vi "FlexMag - 23-03-2023.vi"() -> ()   [LabVIEW 2018] (continued)
                                n19635 = case shown="False" w23986 {
                                frame False {
                                n19636 = local read "coating start"() -> (w23987:bool)
                                n19637 = case shown="True" w23987 {
                                frame False {
                                }
                                frame True {
                                n19638 = while {
                                i -> [w23990]
                                stop <- w23992 stop-if-true
                                n19639 = Greater Or Equal?(x=w23990, y=100) -> (x >= y?=w23991:bool)
                                n19640 = case shown="True" w23991 {
                                frame False {
                                }
                                frame True {
                                n19641 = local write "coating error"(TRUE ("coating error")) -> ()
                                n19642 = local write "Warning Message"("Automatic Coating Process is canceled !\nDCPS Problem.." ("Warning Message")) -> ()
                                }
                                }
                                n19643 = local read "Dcps_fail"() -> (w23996:bool)
                                n19644 = case shown="True" w23996 {
                                tunnel: [TRUE ("CH2_WFC_DO") FALSE ("CH2_WFC_DO")] -> w23995
                                frame False {
                                }
                                frame True {
                                n19645 = Wait Until Next ms Multiple(millisecond multiple=u32 200) -> ()  [unwired: 1 out]
                                }
                                }
                                n19646 = local read "coating start"() -> (w23994:bool)
                                n19647 = local read "abort ch2"() -> (w23988:bool)
                                n19648 = Not(x=w23994) -> (.not. x?=w23993:bool)
                                n19649 = Compound Arithmetic op=OR(w23995, w23993, w23988) -> (w23992:bool)
                                }
                                }
                                }
                                }
                                frame True {
                                }
                                }
                                }
                                frame #2 {
                                n19650 = local read "abort ch2"() -> (w24002:bool)
                                n19651 = case shown="False" w24002 {
                                frame False {
                                n19652 = local read "coating start"() -> (w24003:bool)
                                n19653 = case shown="True" w24003 {
                                frame False {
                                }
                                frame True {
                                n19654 = Wait (ms)(milliseconds to wait=u32 100) -> ()  [unwired: 1 out]
                                "coating ch2 led 4" <- TRUE ("coating ch2 led 1")
                                }
                                }
                                }
                                frame True {
                                }
                                }
                                }
                                }
                                }
                                frame #5 {
                                # "magnetron selection"
                                n19655 = stacked-sequence {
                                frame #0 {
                                n19656 = local read "abort ch2"() -> (w24006:bool)
                                n19657 = case shown="False" w24006 {
                                frame False {
                                n19658 = local read "coating start"() -> (w24007:bool)
                                n19659 = case shown="True" w24007 {
                                frame False {
                                }
                                frame True {
                                n19660 = local write "DCPS_ SW2 DO"(FALSE ("pcgv2 auto open")) -> ()
                                n19661 = local write "DCPS_ SW1 DO"(TRUE ("pcgv2 auto open")) -> ()
                                n19662 = Wait (ms)(milliseconds to wait=u32 1000) -> ()  [unwired: 1 out]
                                }
                                }
                                }
                                frame True {
                                }
                                }
                                }
                                frame #1 {
                                n19663 = local read "abort ch2"() -> (w24011:bool)
                                n19664 = case shown="False" w24011 {
                                frame False {
                                n19665 = local read "coating start"() -> (w24012:bool)
                                n19666 = case shown="True" w24012 {
                                frame False {
                                }
                                frame True {
                                n19667 = while {
                                i -> [w24015]
                                stop <- w24017 stop-if-true
                                n19668 = Greater Or Equal?(x=w24015, y=100) -> (x >= y?=w24016:bool)
                                n19669 = case shown="True" w24016 {
                                frame False {
                                }
                                frame True {
                                n19670 = local write "Warning Message"("Automatic Coating Process is canceled !\nDCPS Magnetron Selection Problem.." ("Warning Message")) -> ()
                                n19671 = local write "coating error"(TRUE ("coating error")) -> ()
                                }
                                }
                                n19672 = local read "DCPS_ SW1 DI"() -> (w24021:bool)
                                n19673 = case shown="False" w24021 {
                                tunnel: [FALSE ("CH2_WFC_DO") TRUE ("CH2_WFC_DO")] -> w24020
                                frame False {
                                n19674 = local write "DCPS_ SW1 DO"(TRUE ("CH2_WFC_DO")) -> ()
                                n19675 = local write "DCPS_ SW2 DO"(FALSE ("CH2_WFC_DO")) -> ()
                                n19676 = Wait Until Next ms Multiple(millisecond multiple=u32 200) -> ()  [unwired: 1 out]
                                }
                                frame True {
                                }
                                }
                                n19677 = local read "coating start"() -> (w24019:bool)
                                n19678 = local read "abort ch2"() -> (w24013:bool)
                                n19679 = Not(x=w24019) -> (.not. x?=w24018:bool)
                                n19680 = Compound Arithmetic op=OR(w24020, w24018, w24013) -> (w24017:bool)
                                }
                                }
                                }
                                }
                                frame True {
                                }
                                }
                                }
                                frame #2 {
                                n19681 = local read "abort ch2"() -> (w24029:bool)
                                n19682 = case shown="False" w24029 {
                                frame False {
                                n19683 = local read "coating start"() -> (w24030:bool)
                                n19684 = case shown="True" w24030 {
                                frame False {
                                }
                                frame True {
                                n19685 = Wait (ms)(milliseconds to wait=u32 100) -> ()  [unwired: 1 out]
                                "coating ch2 led 5" <- TRUE ("coating ch2 led 1")
                                }
                                }
                                }
                                frame True {
                                }
                                }
                                }
                                }
                                }
                                frame #6 {
                                # "cc close"
                                n19686 = stacked-sequence {
                                frame #0 {
                                n19687 = local read "abort ch2"() -> (w24033:bool)
                                n19688 = case shown="False" w24033 {
                                frame False {
                                n19689 = local read "coating start"() -> (w24034:bool)
                                n19690 = case shown="True" w24034 {
                                frame False {
                                }
                                frame True {
                                n19691 = while {
                                i -> [w24037]
                                stop <- w24039 stop-if-true
                                n19692 = Greater Or Equal?(x=w24037, y=100) -> (x >= y?=w24038:bool)
                                n19693 = case shown="True" w24038 {
                                frame False {
                                }
                                frame True {
                                n19694 = local write "Warning Message"("Automatic Coating Process is canceled !\nCH2 ColdCathode couldn't be closed.." ("Warning Message")) -> ()
                                n19695 = local write "coating error"(TRUE ("coating error")) -> ()
                                }
                                }
                                n19696 = local read "CH2_CC_DI"() -> (w24043:bool)
                                n19697 = case shown="True" w24043 {
                                tunnel: [TRUE ("CH2_WFC_DO") FALSE ("CH2_WFC_DO")] -> w24042
                                frame False {
                                }
                                frame True {
                                n19698 = Wait Until Next ms Multiple(millisecond multiple=u32 200) -> ()  [unwired: 1 out]
                                n19699 = local write "CH2_CC_DO"(FALSE ("coating error")) -> ()
                                }
                                }
                                n19700 = local read "coating start"() -> (w24041:bool)
                                n19701 = local read "abort ch2"() -> (w24035:bool)
                                n19702 = Not(x=w24041) -> (.not. x?=w24040:bool)
                                n19703 = Compound Arithmetic op=OR(w24042, w24040, w24035) -> (w24039:bool)
                                }
                                }
                                }
                                }
                                frame True {
                                }
                                }
                                }
                                frame #1 {
                                n19704 = local read "abort ch2"() -> (w24050:bool)
                                n19705 = case shown="False" w24050 {
                                frame False {
                                n19706 = local read "coating start"() -> (w24051:bool)
                                n19707 = case shown="True" w24051 {
                                frame False {
                                }
                                frame True {
                                n19708 = Wait (ms)(milliseconds to wait=u32 100) -> ()  [unwired: 1 out]
                                "coating ch2 led 6" <- TRUE ("coating ch2 led 1")
                                }
                                }
                                }
                                frame True {
                                }
                                }
                                }
                                }
                                }
                                frame #7 {
                                # "baratron bv open"
                                n19709 = stacked-sequence {
                                frame #0 {
                                n19710 = local read "abort ch2"() -> (w24054:bool)
                                n19711 = case shown="False" w24054 {
                                frame False {
                                n19712 = local read "coating start"() -> (w24055:bool)
                                n19713 = case shown="True" w24055 {
                                frame False {
                                }
                                frame True {
                                n19714 = while {
                                i -> [w24058]
                                stop <- w24060 stop-if-true
                                n19715 = Greater Or Equal?(x=w24058, y=100) -> (x >= y?=w24059:bool)
                                n19716 = case shown="True" w24059 {
                                frame False {
                                }
                                frame True {
                                n19717 = local write "Warning Message"("Automatic Coating Process is canceled !\nCH2 Baratron Gauge Block Valve couldn't be opned.." ("Warning Message")) -> ()
                                n19718 = local write "coating error"(TRUE ("coating error")) -> ()
                                }
                                }
                                n19719 = local read "CH2_BG_BV_DI"() -> (w24064:bool)
                                n19720 = case shown="False" w24064 {
                                tunnel: [FALSE ("CH2_WFC_DO") TRUE ("CH2_WFC_DO")] -> w24063
                                frame False {
                                n19721 = Wait Until Next ms Multiple(millisecond multiple=u32 200) -> ()  [unwired: 1 out]
                                n19722 = local write "CH2_BG_BV_DO"(TRUE ("coating error")) -> ()
                                }
                                frame True {
                                }
                                }
                                n19723 = local read "coating start"() -> (w24062:bool)
                                n19724 = local read "abort ch2"() -> (w24056:bool)
                                n19725 = Not(x=w24062) -> (.not. x?=w24061:bool)
                                n19726 = Compound Arithmetic op=OR(w24063, w24061, w24056) -> (w24060:bool)
                                }
                                }
                                }
                                }
                                frame True {
                                }
                                }
                                }
                                frame #1 {
                                n19727 = local read "abort ch2"() -> (w24071:bool)
                                n19728 = case shown="False" w24071 {
                                frame False {
                                n19729 = local read "coating start"() -> (w24072:bool)
                                n19730 = case shown="True" w24072 {
                                frame False {
                                }
                                frame True {
                                n19731 = Wait (ms)(milliseconds to wait=u32 100) -> ()  [unwired: 1 out]
                                "coating ch2 led 7" <- TRUE ("coating ch2 led 1")
                                }
                                }
                                }
                                frame True {
                                }
                                }
                                }
                                }
                                }
                                frame #8 {
                                # "ar sov open"
                                n19732 = stacked-sequence {
                                frame #0 {
                                n19733 = local read "abort ch2"() -> (w24075:bool)
                                n19734 = case shown="False" w24075 {
                                frame False {
                                n19735 = local read "coating start"() -> (w24076:bool)
                                n19736 = case shown="True" w24076 {
                                frame False {
                                }
                                frame True {
                                n19737 = while {
                                i -> [w24079]
                                stop <- w24081 stop-if-true
                                n19738 = Greater Or Equal?(x=w24079, y=100) -> (x >= y?=w24080:bool)
                                n19739 = case shown="True" w24080 {
                                frame False {
                                }
                                frame True {
                                n19740 = local write "Warning Message"("Automatic Coating Process is canceled !\nCH2 SoV Ar couldn't be opened.." ("Warning Message")) -> ()
                                n19741 = local write "coating error"(TRUE ("coating error")) -> ()
                                }
                                }
                                n19742 = local read "CH2_SoV_Ar_DI"() -> (w24085:bool)
                                n19743 = case shown="False" w24085 {
                                tunnel: [FALSE ("CH2_WFC_DO") TRUE ("CH2_WFC_DO")] -> w24084
                                frame False {
                                n19744 = Wait Until Next ms Multiple(millisecond multiple=u32 200) -> ()  [unwired: 1 out]
                                n19745 = local write "CH2_SoV_Ar_DO"(TRUE ("coating error")) -> ()
                                }
                                frame True {
                                }
                                }
                                n19746 = local read "coating start"() -> (w24083:bool)
                                n19747 = local read "abort ch2"() -> (w24077:bool)
                                n19748 = Not(x=w24083) -> (.not. x?=w24082:bool)
                                n19749 = Compound Arithmetic op=OR(w24084, w24082, w24077) -> (w24081:bool)
                                }
                                }
                                }
                                }
                                frame True {
                                }
                                }
                                }
                                frame #1 {
                                n19750 = local read "abort ch2"() -> (w24092:bool)
                                n19751 = case shown="False" w24092 {
                                frame False {
                                n19752 = local read "coating start"() -> (w24093:bool)
                                n19753 = case shown="True" w24093 {
                                frame False {
                                }
                                frame True {
                                n19754 = Wait (ms)(milliseconds to wait=u32 100) -> ()  [unwired: 1 out]
                                "coating ch2 led 8" <- TRUE ("coating ch2 led 1")
                                }
                                }
                                }
                                frame True {
                                }
                                }
                                }
                                }
                                }
                                frame #9 {
                                # "mfc set"
                                n19755 = stacked-sequence {
                                frame #0 {
                                n19756 = local read "abort ch2"() -> (w24096:bool)
                                n19757 = case shown="False" w24096 {
                                frame False {
                                n19758 = local read "coating start"() -> (w24097:bool)
                                n19759 = case shown="True" w24097 {
                                frame False {
                                }
                                frame True {
                                n19760 = flat-sequence {
                                frame #0 {
                                n19761 = local read "R Ar set sccm"() -> (w24099:dbl)
                                n19762 = local write "ch2 argon mfc set"(w24099) -> ()
                                n19763 = Wait (ms)(milliseconds to wait=u32 300) -> ()  [unwired: 1 out]
                                }
                                frame #1 {
                                n19764 = local write "ch2 ar set auto"(TRUE ("ch2 ar set auto")) -> ()
                                }
                                }
                                }
                                }
                                }
                                frame True {
                                }
                                }
                                }
                                frame #1 {
                                n19765 = local read "abort ch2"() -> (w24101:bool)
                                n19766 = case shown="False" w24101 {
                                frame False {
                                n19767 = local read "coating start"() -> (w24102:bool)
                                n19768 = case shown="True" w24102 {
                                frame False {
                                }
                                frame True {
                                n19769 = while {
                                i -> [w24112]
                                stop <- w24114 stop-if-true
                                n19770 = local read "R Ar set sccm"() -> (w24108:dbl)
                                n19771 = Greater Or Equal?(x=w24112, y=50) -> (x >= y?=w24113:bool)
                                n19772 = case shown="True" w24113 {
                                frame False {
                                }
                                frame True {
                                n19773 = local write "Warning Message"("Automatic Coating Process is canceled !\nCH2  MFC Ar flow problem..." ("Warning Message")) -> ()
                                n19774 = local write "coating error"(TRUE ("coating error")) -> ()
                                }
                                }
                                n19775 = local read "ch2 argon mfc actual"() -> (w24109:dbl)
                                n19776 = Add(x=w24108, y=5.0) -> (x+y=w24105:dbl)
                                n19777 = Subtract(x=w24108, y=5.0) -> (x-y=w24104:dbl)
                                n19778 = In Range and Coerce(upper limit=w24105, x=w24109, lower limit=w24104) -> (In Range?=w24103:bool)  [unwired: 1 out]
                                n19779 = case shown="False" w24103 {
                                tunnel: [FALSE ("CH2_WFC_DO") TRUE ("CH2_WFC_DO")] -> w24117
                                frame False {
                                n19780 = Wait Until Next ms Multiple(millisecond multiple=u32 1000) -> ()  [unwired: 1 out]
                                n19781 = local write "ch2 ar set auto"(TRUE ("coating error")) -> ()
                                }
                                frame True {
                                }
                                }
                                n19782 = local read "coating start"() -> (w24116:bool)
                                n19783 = local read "abort ch2"() -> (w24110:bool)
                                n19784 = Not(x=w24116) -> (.not. x?=w24115:bool)
                                n19785 = Compound Arithmetic op=OR(w24117, w24115, w24110) -> (w24114:bool)
                                }
                                }
                                }
                                }
                                frame True {
                                }
                                }
                                }
                                frame #2 {
                                n19786 = local read "abort ch2"() -> (w24124:bool)
                                n19787 = case shown="False" w24124 {
                                frame False {
                                n19788 = local read "coating start"() -> (w24125:bool)
                                n19789 = case shown="True" w24125 {
                                frame False {
                                }
                                frame True {
                                n19790 = Wait (ms)(milliseconds to wait=u32 100) -> ()  [unwired: 1 out]
                                "coating ch2 led 9" <- TRUE ("coating ch2 led 1")
                                }
                                }
                                }
                                frame True {
                                }
                                }
                                }
                                }
                                }
                                frame #10 {
                                # "baratron pressure set"
                                n19791 = stacked-sequence {
                                frame #0 {
                                n19792 = local read "abort ch2"() -> (w24128:bool)
                                n19793 = case shown="False" w24128 {
                                frame False {
                                n19794 = local read "coating start"() -> (w24129:bool)
                                n19795 = case shown="True" w24129 {
                                frame False {
                                }
                                frame True {
                                n19796 = flat-sequence {
                                frame #0 {
                                n19797 = local read "R Pressure set mbar"() -> (w24130:dbl)
                                n19798 = Wait (ms)(milliseconds to wait=u32 300) -> ()  [unwired: 1 out]
                                n19799 = local write "pcgv2 set pressure value mbar"(w24130) -> ()
                                }
                                frame #1 {
                                n19800 = local write "pcgv2 auto set pressure"(TRUE ("ch2 ar set auto")) -> ()
                                }
                                }
                                }
                                }
                                }
                                frame True {
                                }
                                }
                                }
                                frame #1 {
                                n19801 = local read "abort ch2"() -> (w24133:bool)
                                n19802 = case shown="False" w24133 {
                                frame False {
                                n19803 = local read "coating start"() -> (w24134:bool)
                                n19804 = case shown="True" w24134 {
                                frame False {
                                }
                                frame True {
                                n19805 = while {
                                i -> [w24144]
                                stop <- w24146 stop-if-true
                                n19806 = local read "R Pressure set mbar"() -> (w24140:dbl)
                                n19807 = Greater Or Equal?(x=w24144, y=50) -> (x >= y?=w24145:bool)
                                n19808 = case shown="True" w24145 {
                                frame False {
                                }
                                frame True {
                                n19809 = local write "Warning Message"("Automatic Coating Process is canceled !\nCH2 Baratron Pressure Set problem..." ("Warning Message")) -> ()
                                n19810 = local write "coating error"(TRUE ("coating error")) -> ()
                                }
                                }
                                n19811 = local read "Ch2_baratron_pressure_mbar"() -> (w24141:dbl)
                                n19812 = Add(x=w24140, y=0.003) -> (x+y=w24137:dbl)
                                n19813 = Subtract(x=w24140, y=0.003) -> (x-y=w24136:dbl)
                                n19814 = In Range and Coerce(upper limit=w24137, x=w24141, lower limit=w24136) -> (In Range?=w24135:bool)  [unwired: 1 out]
                                n19815 = case shown="False" w24135 {
                                tunnel: [FALSE ("CH2_WFC_DO") TRUE ("CH2_WFC_DO")] -> w24149
                                frame False {
                                n19816 = Wait Until Next ms Multiple(millisecond multiple=u32 1000) -> ()  [unwired: 1 out]
                                n19817 = local write "pcgv2 auto set pressure"(TRUE ("coating error")) -> ()
                                }
                                frame True {
                                }
                                }
                                n19818 = local read "coating start"() -> (w24148:bool)
                                n19819 = local read "abort ch2"() -> (w24142:bool)
                                n19820 = Not(x=w24148) -> (.not. x?=w24147:bool)
                                n19821 = Compound Arithmetic op=OR(w24149, w24147, w24142) -> (w24146:bool)
                                }
                                }
                                }
                                }
                                frame True {
                                }
                                }
                                }
                                frame #2 {
                                n19822 = local read "abort ch2"() -> (w24156:bool)
                                n19823 = case shown="False" w24156 {
                                frame False {
                                n19824 = local read "coating start"() -> (w24157:bool)
                                n19825 = case shown="True" w24157 {
                                frame False {
                                }
                                frame True {
                                n19826 = Wait (ms)(milliseconds to wait=u32 100) -> ()  [unwired: 1 out]
                                "coating ch2 led 10" <- TRUE ("coating ch2 led 1")
                                }
                                }
                                }
                                frame True {
                                }
                                }
                                }
                                }
                                }
                                frame #11 {
                                # "power set"
                                n19827 = stacked-sequence {
                                frame #0 {
                                n19828 = local read "abort ch2"() -> (w24160:bool)
                                n19829 = case shown="False" w24160 {
                                frame False {
                                n19830 = local read "coating start"() -> (w24161:bool)
                                n19831 = case shown="True" w24161 {
                                frame False {
                                }
                                frame True {
                                n19832 = flat-sequence {
                                frame #0 {
                                n19833 = local write "Dc_auto_off"(TRUE ("Dc_auto_off")) -> ()
                                }
                                frame #1 {
                                # "200 watt is good to ignite plasma"
                                n19834 = local write "Set DC Power auto"(200.0 ("Set DC Power")) -> ()
                                n19835 = Wait (ms)(milliseconds to wait=u32 2000) -> ()  [unwired: 1 out]
                                }
                                frame #2 {
                                n19836 = local write "Dc_auto_set"(TRUE ("Dc_auto_set")) -> ()
                                }
                                }
                                }
                                }
                                }
                                frame True {
                                }
                                }
                                }
                                frame #1 {
                                n19837 = local read "abort ch2"() -> (w24166:bool)
                                n19838 = case shown="False" w24166 {
                                frame False {
                                n19839 = local read "coating start"() -> (w24167:bool)
                                n19840 = case shown="True" w24167 {
                                frame False {
                                }
                                frame True {
                                n19841 = flat-sequence {
                                frame #0 {
                                n19842 = local read "R web thickness"() -> (w24182:dbl)
                                n19843 = local read "R core diameter"() -> (w24183:dbl)
                                n19844 = local read "R tension value"() -> (w24181:dbl)
                                n19845 = local read "R dc step length 10"() -> (w24171:dbl)
                                n19846 = local read "R web speed"() -> (w24168:dbl)
                                n19847 = local read "R dc step length 1"() -> (w24180:dbl)
                                n19848 = local read "R dc step length 2"() -> (w24179:dbl)
                                n19849 = local read "R dc step length 3"() -> (w24178:dbl)
                                n19850 = local read "R dc step length 4"() -> (w24177:dbl)
                                n19851 = local read "R dc step length 5"() -> (w24176:dbl)
                                n19852 = local read "R dc step length 6"() -> (w24175:dbl)
                                n19853 = local read "R dc step length 7"() -> (w24174:dbl)
                                n19854 = local read "R dc step length 8"() -> (w24173:dbl)
                                n19855 = local read "R dc step length 9"() -> (w24172:dbl)
                                n19856 = local write "web speed"(w24168) -> ()
                                n19857 = local write "initial right diameter"(w24183) -> ()
                                n19858 = local write "web thickness"(w24182) -> ()
                                n19859 = local write "tension value"(w24181) -> ()
                                n19860 = local write "setpoint"(w24168) -> ()
                                n19861 = Compound Arithmetic op=ADD(w24180, w24179, w24178, w24177, w24176, w24175, w24174, w24173, w24172, w24171) -> (w24170:dbl)
                                n19862 = local write "target interval"(w24170) -> ()
                                n19863 = Wait (ms)(milliseconds to wait=u32 500) -> ()  [unwired: 1 out]
                                }
                                frame #1 {
                                n19864 = Wait (ms)(milliseconds to wait=u32 500) -> ()  [unwired: 1 out]
                                }
                                frame #2 {
                                n19865 = local write "calculate"(TRUE ("calculate")) -> ()
                                }
                                }
                                }
                                }
                                }
                                frame True {
                                }
                                }
                                }
                                frame #2 {
                                n19866 = local read "abort ch2"() -> (w24186:bool)
                                n19867 = case shown="False" w24186 {
                                frame False {
                                n19868 = local read "coating start"() -> (w24187:bool)
                                n19869 = case shown="True" w24187 {
                                frame False {
                                }
                                frame True {
                                n19870 = flat-sequence {
                                frame #0 {
                                n19871 = while {
                                i -> [w24192]
                                stop <- w24188 stop-if-true
                                n19872 = local read "coating start"() -> (w24196:bool)
                                n19873 = local read "calculate"() -> (w24197:bool)
                                n19874 = local read "abort ch2"() -> (w24195:bool)
                                n19875 = Greater Or Equal?(x=w24192, y=60) -> (x >= y?=w24189:bool)
                                n19876 = Not(x=w24197) -> (.not. x?=w24193:bool)
                                n19877 = Not(x=w24196) -> (.not. x?=w24194:bool)
                                n19878 = Wait Until Next ms Multiple(millisecond multiple=u32 1000) -> ()  [unwired: 1 out]
                                n19879 = Compound Arithmetic op=OR(w24189, w24193, w24194, w24195) -> (w24188:bool)
                                }
                                }
                                frame #1 {
                                n19880 = local read "R DC number steps"() -> (w24199:dbl)
                                n19881 = Wait (ms)(milliseconds to wait=u32 1000) -> ()  [unwired: 1 out]
                                n19882 = local write "current step"(0.0 ("step count")) -> ()
                                n19883 = local write "step count"(w24199) -> ()
                                }
                                }
                                }
                                }
                                }
                                frame True {
                                }
                                }
                                }
                                frame #3 {
                                n19884 = local read "abort ch2"() -> (w24201:bool)
                                n19885 = case shown="False" w24201 {
                                frame False {
                                n19886 = local read "coating start"() -> (w24202:bool)
                                n19887 = case shown="True" w24202 {
                                frame False {
                                }
                                frame True {
                                n19888 = flat-sequence {
                                frame #0 {
                                n19889 = local read "dep. for?"() -> (w24203:bool)
                                n19890 = case shown="False" w24203 {
                                frame False {
                                n19891 = local write "back roll"(TRUE ("back roll")) -> ()
                                }
                                frame True {
                                n19892 = local write "forward roll"(TRUE ("forward roll")) -> ()
                                }
                                }
                                }
                                frame #1 {
                                n19893 = Wait (ms)(milliseconds to wait=u32 1000) -> ()  [unwired: 1 out]
                                }
                                frame #2 {
                                n19894 = while {
                                i -> [w24212]
                                stop <- w24209 stop-if-true
                                n19895 = local read "CH2_Motor DO"() -> (w24208:bool)
                                n19896 = local read "coating start"() -> (w24215:bool)
                                n19897 = local read "abort ch2"() -> (w24214:bool)
                                n19898 = Greater Or Equal?(x=w24212, y=60) -> (x >= y?=w24207:bool)
                                n19899 = Wait Until Next ms Multiple(millisecond multiple=u32 1000) -> ()  [unwired: 1 out]
                                n19900 = Not(x=w24215) -> (.not. x?=w24213:bool)
                                n19901 = local write "Dc_auto_on"(w24208) -> ()
                                n19902 = Compound Arithmetic op=OR(w24208, w24213, w24214, w24207) -> (w24209:bool)
                                n19903 = local write "coating error"(w24207) -> ()
                                }
                                }
                                frame #3 {
                                n19904 = Wait (ms)(milliseconds to wait=u32 500) -> ()  [unwired: 1 out]
                                }
                                }
                                }
                                }
                                }
                                frame True {
                                }
                                }
                                }
                                frame #4 {
                                n19905 = local read "abort ch2"() -> (w24217:bool)
                                n19906 = case shown="False" w24217 {
                                frame False {
                                n19907 = local read "coating start"() -> (w24218:bool)
                                n19908 = case shown="True" w24218 {
                                frame False {
                                }
                                frame True {
                                }
                                }
                                }
                                frame True {
                                }
                                }
                                }
                                frame #5 {
                                n19909 = local read "abort ch2"() -> (w24219:bool)
                                n19910 = case shown="False" w24219 {
                                frame False {
                                n19911 = local read "coating start"() -> (w24220:bool)
                                n19912 = case shown="True" w24220 {
                                frame False {
                                }
                                frame True {
                                n19913 = Wait (ms)(milliseconds to wait=u32 100) -> ()  [unwired: 1 out]
                                "coating ch2 led 11" <- TRUE ("coating ch2 led 1")
                                }
                                }
                                }
                                frame True {
                                }
                                }
                                }
                                }
                                }
                                frame #12 {
                                # "power steps"
                                n19914 = disable-structure shown="Enabled" {
                                frame Disabled {
                                n19915 = stacked-sequence {
                                frame #0 {
                                n19916 = local read "abort ch2"() -> (w24223:bool)
                                n19917 = case shown="False" w24223 {
                                frame False {
                                n19918 = local read "coating start"() -> (w24224:bool)
                                n19919 = case shown="True" w24224 {
                                frame False {
                                }
                                frame True {
                                n19920 = local read "R dc step length 1"() -> (w24227:dbl)
                                n19921 = Greater?(x=w24227, y=0.0) -> (0:w24226:bool)
                                n19922 = case shown="True" w24226 {
                                frame False {
                                }
                                frame True {
                                n19923 = flat-sequence {
                                frame #0 {
                                n19924 = local read "R dc step length 1"() -> (w24234:dbl)
                                n19925 = local read "R dc step power 1"() -> (w24229:dbl)
                                n19926 = local read "R web speed"() -> (w24233:dbl)
                                n19927 = Divide(x=w24234, y=w24233) -> (x/y=w24232:dbl)
                                n19928 = local write "Set DC Power ch2"(w24229) -> ()
                                n19929 = Multiply(x=w24232, y=60) -> (x*y=w24230:dbl)
                                n19930 = Wait (ms)(milliseconds to wait=u32 100) -> ()  [unwired: 1 out]
                                n19931 = local write "time counting"(w24230) -> ()
                                }
                                frame #1 {
                                n19932 = local write "Dc_auto_set"(TRUE ("Dc_auto_set")) -> ()
                                }
                                frame #2 {
                                n19933 = while {
                                stop <- w24237 stop-if-true
                                n19934 = local read "time counting"() -> (w24243:dbl)
                                n19935 = Wait Until Next ms Multiple(millisecond multiple=u32 1000) -> ()  [unwired: 1 out]
                                n19936 = local read "coating start"() -> (w24241:bool)
                                n19937 = local read "abort ch2"() -> (w24239:bool)
                                n19938 = Decrement(x=w24243) -> (x-1=w24242:dbl)
                                n19939 = local write "time counting"(w24242) -> ()
                                n19940 = Not(x=w24241) -> (.not. x?=w24240:bool)
                                n19941 = Less Or Equal To 0?(x=w24242) -> (x <= 0?=w24238:bool)
                                n19942 = Compound Arithmetic op=OR(w24238, w24240, w24239) -> (w24237:bool)
                                }
                                }
                                }
                                }
                                }
                                }
                                }
                                }
                                frame True {
                                }
                                }
                                }
                                frame #1 {
                                n19943 = local read "abort ch2"() -> (w24244:bool)
                                n19944 = case shown="False" w24244 {
                                frame False {
                                n19945 = local read "coating start"() -> (w24245:bool)
                                n19946 = case shown="True" w24245 {
                                frame False {
                                }
                                frame True {
                                n19947 = local read "R dc step length 2"() -> (w24248:dbl)
                                n19948 = Greater?(x=w24248, y=0.0) -> (0:w24247:bool)
                                n19949 = case shown="True" w24247 {
                                frame False {
                                }
                                frame True {
                                n19950 = flat-sequence {
                                frame #0 {
                                n19951 = local read "R dc step length 2"() -> (w24255:dbl)
                                n19952 = local read "R dc step power 2"() -> (w24250:dbl)
                                n19953 = local read "R web speed"() -> (w24254:dbl)
                                n19954 = Divide(x=w24255, y=w24254) -> (x/y=w24253:dbl)
                                n19955 = local write "Set DC Power ch2"(w24250) -> ()
                                n19956 = Multiply(x=w24253, y=60) -> (x*y=w24251:dbl)
                                n19957 = Wait (ms)(milliseconds to wait=u32 100) -> ()  [unwired: 1 out]
                                n19958 = local write "time counting"(w24251) -> ()
                                }
                                frame #1 {
                                n19959 = local write "Dc_auto_set"(TRUE ("Dc_auto_set")) -> ()
                                }
                                frame #2 {
                                n19960 = while {
                                stop <- w24258 stop-if-true
                                n19961 = local read "time counting"() -> (w24264:dbl)
                                n19962 = local read "coating start"() -> (w24262:bool)
                                n19963 = local read "abort ch2"() -> (w24260:bool)
                                n19964 = Wait Until Next ms Multiple(millisecond multiple=u32 1000) -> ()  [unwired: 1 out]
                                n19965 = Decrement(x=w24264) -> (x-1=w24263:dbl)
                                n19966 = local write "time counting"(w24263) -> ()
                                n19967 = Not(x=w24262) -> (.not. x?=w24261:bool)
                                n19968 = Less Or Equal To 0?(x=w24263) -> (x <= 0?=w24259:bool)
                                n19969 = Compound Arithmetic op=OR(w24259, w24261, w24260) -> (w24258:bool)
                                }
                                }
                                }
                                }
                                }
                                }
                                }
                                }
                                frame True {
                                }
                                }
                                }
                                frame #2 {
                                n19970 = local read "abort ch2"() -> (w24265:bool)
                                n19971 = case shown="False" w24265 {
                                frame False {
                                n19972 = local read "coating start"() -> (w24266:bool)
                                n19973 = case shown="True" w24266 {
                                frame False {
                                }
                                frame True {
                                n19974 = local read "R dc step length 3"() -> (w24269:dbl)
                                n19975 = Greater?(x=w24269, y=0.0) -> (0:w24268:bool)
                                n19976 = case shown="True" w24268 {
                                frame False {
                                }
                                frame True {
                                n19977 = flat-sequence {
                                frame #0 {
                                n19978 = local read "R dc step length 3"() -> (w24276:dbl)
                                n19979 = local read "R dc step power 3"() -> (w24271:dbl)
                                n19980 = local read "R web speed"() -> (w24275:dbl)
                                n19981 = Divide(x=w24276, y=w24275) -> (x/y=w24274:dbl)
                                n19982 = local write "Set DC Power ch2"(w24271) -> ()
                                n19983 = Multiply(x=w24274, y=60) -> (x*y=w24272:dbl)
                                n19984 = Wait (ms)(milliseconds to wait=u32 100) -> ()  [unwired: 1 out]
                                n19985 = local write "time counting"(w24272) -> ()
                                }
                                frame #1 {
                                n19986 = local write "Dc_auto_set"(TRUE ("Dc_auto_set")) -> ()
                                }
                                frame #2 {
                                n19987 = while {
                                stop <- w24279 stop-if-true
                                n19988 = local read "time counting"() -> (w24285:dbl)
                                n19989 = local read "coating start"() -> (w24283:bool)
                                n19990 = Wait Until Next ms Multiple(millisecond multiple=u32 1000) -> ()  [unwired: 1 out]
                                n19991 = local read "abort ch2"() -> (w24281:bool)
                                n19992 = Decrement(x=w24285) -> (x-1=w24284:dbl)
                                n19993 = local write "time counting"(w24284) -> ()
                                n19994 = Not(x=w24283) -> (.not. x?=w24282:bool)
                                n19995 = Less Or Equal To 0?(x=w24284) -> (x <= 0?=w24280:bool)
                                n19996 = Compound Arithmetic op=OR(w24280, w24282, w24281) -> (w24279:bool)
                                }
                                }
                                }
                                }
                                }
                                }
                                }
                                }
                                frame True {
                                }
                                }
                                }
                                frame #3 {
                                n19997 = local read "abort ch2"() -> (w24286:bool)
                                n19998 = case shown="False" w24286 {
                                frame False {
                                n19999 = local read "coating start"() -> (w24287:bool)
                                n20000 = case shown="True" w24287 {
                                frame False {
                                }
                                frame True {
                                n20001 = local read "R dc step length 4"() -> (w24290:dbl)
                                n20002 = Greater?(x=w24290, y=0.0) -> (0:w24289:bool)
                                n20003 = case shown="True" w24289 {
                                frame False {
                                }
                                frame True {
                                n20004 = flat-sequence {
                                frame #0 {
                                n20005 = local read "R dc step length 4"() -> (w24297:dbl)
                                n20006 = local read "R dc step power 4"() -> (w24292:dbl)
                                n20007 = local read "R web speed"() -> (w24296:dbl)
                                n20008 = Divide(x=w24297, y=w24296) -> (x/y=w24295:dbl)
                                n20009 = local write "Set DC Power ch2"(w24292) -> ()
                                n20010 = Wait (ms)(milliseconds to wait=u32 100) -> ()  [unwired: 1 out]
                                n20011 = Multiply(x=w24295, y=60) -> (x*y=w24293:dbl)
                                n20012 = local write "time counting"(w24293) -> ()
                                }
                                frame #1 {
                                n20013 = local write "Dc_auto_set"(TRUE ("Dc_auto_set")) -> ()
                                }
                                frame #2 {
                                n20014 = while {
                                stop <- w24300 stop-if-true
                                n20015 = local read "time counting"() -> (w24306:dbl)
                                n20016 = local read "coating start"() -> (w24304:bool)
                                n20017 = local read "abort ch2"() -> (w24302:bool)
                                n20018 = Wait Until Next ms Multiple(millisecond multiple=u32 1000) -> ()  [unwired: 1 out]
                                n20019 = Decrement(x=w24306) -> (x-1=w24305:dbl)
                                n20020 = local write "time counting"(w24305) -> ()
                                n20021 = Not(x=w24304) -> (.not. x?=w24303:bool)
                                n20022 = Less Or Equal To 0?(x=w24305) -> (x <= 0?=w24301:bool)
                                n20023 = Compound Arithmetic op=OR(w24301, w24303, w24302) -> (w24300:bool)
                                }
                                }
                                }
                                }
                                }
                                }
                                }
                                }
                                frame True {
                                }
                                }
                                }
                                frame #4 {
                                n20024 = local read "abort ch2"() -> (w24307:bool)
                                n20025 = case shown="False" w24307 {
                                frame False {
                                n20026 = local read "coating start"() -> (w24308:bool)
                                n20027 = case shown="True" w24308 {
                                frame False {
                                }
                                frame True {
                                n20028 = local read "R dc step length 5"() -> (w24311:dbl)